vi "H1R_Ref_Pix_Subtract.vi"(9 "Num Ref Pix":i32=5, 11 "Orig Array":i32[][](array[numeric])=array1024x1024[1048576 elements]) -> (3 "Sub Array":i32[][](array[numeric]))   [LabVIEW 2017]
panel:
  out "Q3 avg":dbl=-0.8184616088867186
  out "Q3 RMS":dbl=19.25740971624928
  out "Q4 avg":dbl=1.3942337036132815
  out "Q4 RMS":dbl=26.97344260258525
  out "Q1 RMS":dbl=21.389760464347606
  out "Q1 avg":dbl=2.3578338623046875
  out "Q2  RMS":dbl=28.329968380841386
  out "Q2 avg":dbl=0.05986480712890625
  out "mean before":dbl=0.1424398422241211
  out "RMS before":dbl=23.67379491089448
  out "mean a fter":dbl=0.7448520660400391
  out "RMS  after":dbl=24.28217603569673
  out "IMAGE 2":i32[][](graph)
  out "IMAGE":i32[][](graph)
  in  "Array side Q3":u16(ring)=2 items=["Left", "Bottom", "Right", "Top"]
  in  "Array side Q4":u16(ring)=2 items=["Left", "Bottom", "Right", "Top"]
  in  "Array side Q1":u16(ring) items=["Left", "Bottom", "Right", "Top"]
  in  "Array side Q2":u16(ring) items=["Left", "Bottom", "Right", "Top"]
  # "right"
  # "left"
  # "left"
  # "right"
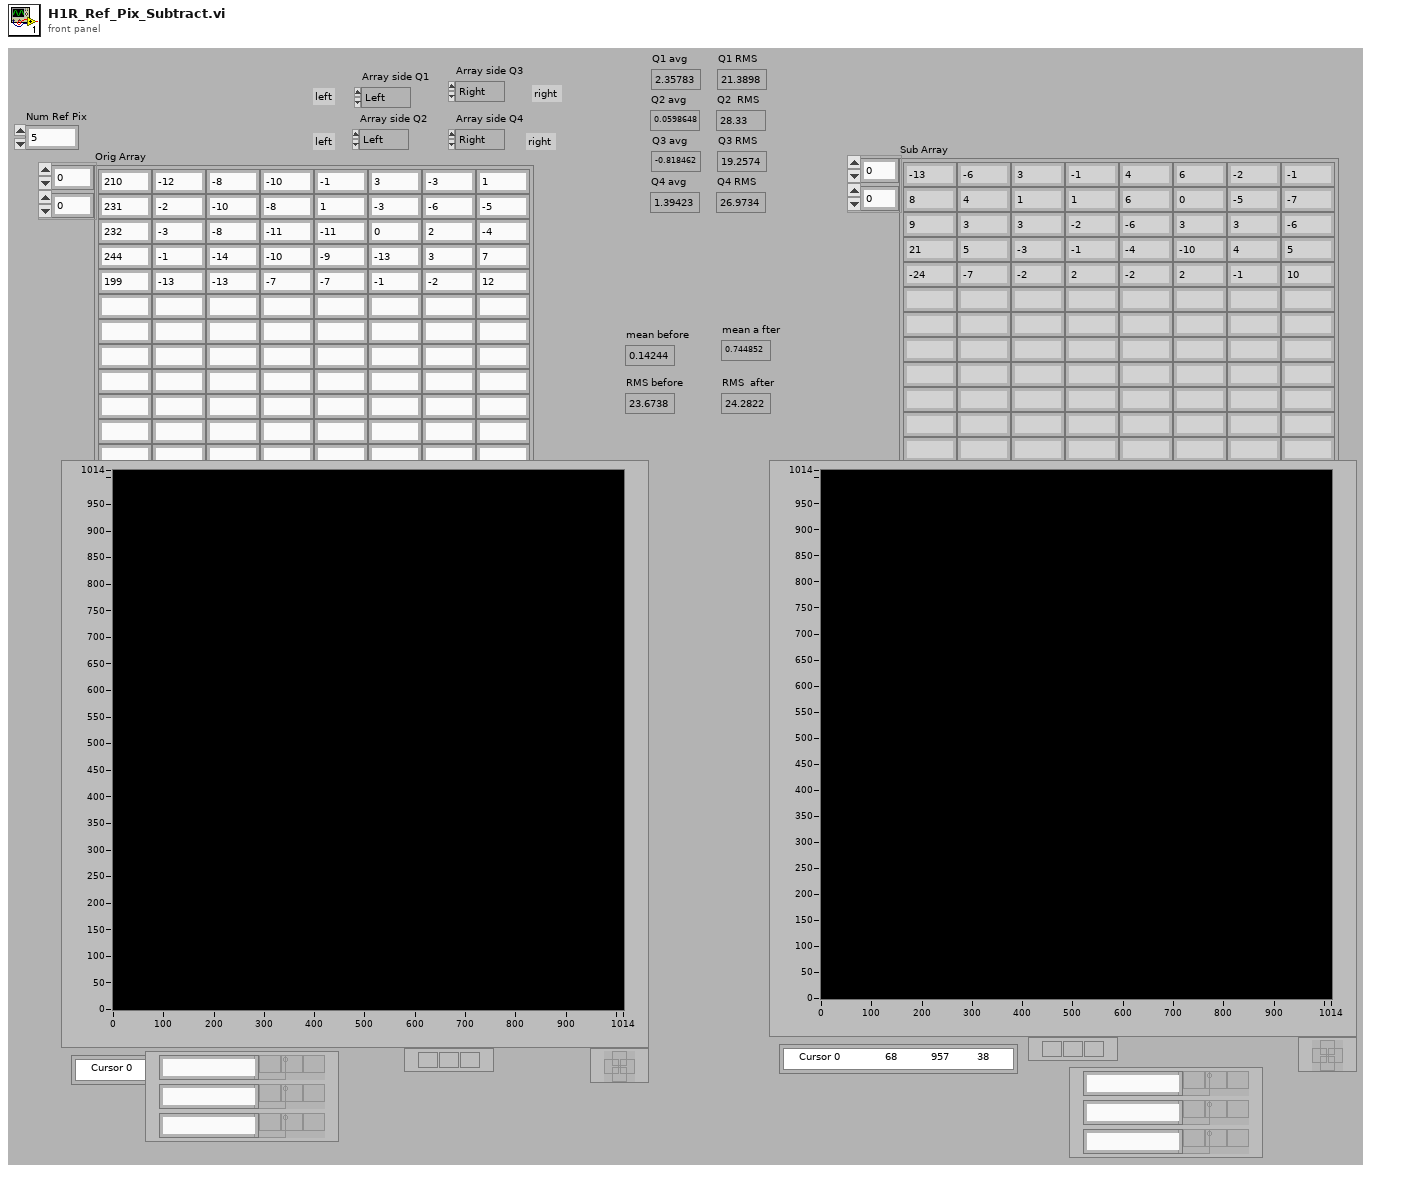
[diagram p1: front panel]
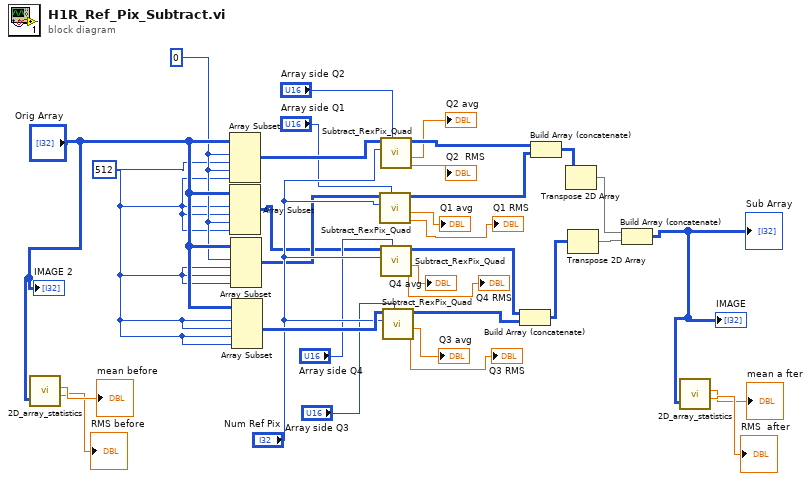
[diagram p0: block diagram]
diagram:
  w4 = 0
  w1 = 512
  n1 = call <userlib>:"2D_array_statistics.vi"("Array"="Orig Array") -> ("mean 2"=→"mean before":dbl, "RMS 2"=→"RMS before":dbl)  [unwired: 2 in, 2 out]
  n2 = Array Subset(array="Orig Array", index (row)=w4, length (row)=w1, index (col)=w4, length (col)=w1) -> (w29:i32[][])
  n3 = Array Subset(array="Orig Array", index (row)=w1, length (row)=w1, index (col)=w4, length (col)=w1) -> (w2:i32[][])
  n4 = Array Subset(array="Orig Array", index (row)=w4, length (row)=w1, index (col)=w1, length (col)=w1) -> (w3:i32[][])
  n5 = Array Subset(array="Orig Array", index (row)=w1, length (row)=w1, index (col)=w1, length (col)=w1) -> (w27:i32[][])
  n6 = call <userlib>:"Subtract_RexPix_Quad.vi"("Array side"="Array side Q1", "Num Ref Pix"="Num Ref Pix", "Quad array"=w3) -> ("RMS 2"=→"Q1 RMS":dbl, "mean 2"=→"Q1 avg":dbl, "Quad array subtracted ref pixs"=w25:i32[][])  [unwired: 5 in, 1 out]
  n7 = call <userlib>:"Subtract_RexPix_Quad.vi"("Array side"="Array side Q2", "Num Ref Pix"="Num Ref Pix", "Quad array"=w29) -> ("RMS 2"=→"Q2  RMS":dbl, "mean 2"=→"Q2 avg":dbl, "Quad array subtracted ref pixs"=w28:i32[][])  [unwired: 5 in, 1 out]
  n8 = call <userlib>:"Subtract_RexPix_Quad.vi"("Array side"="Array side Q4", "Num Ref Pix"="Num Ref Pix", "Quad array"=w2) -> ("RMS 2"=→"Q4 RMS":dbl, "mean 2"=→"Q4 avg":dbl, "Quad array subtracted ref pixs"=w24:i32[][])  [unwired: 5 in, 1 out]
  n9 = call <userlib>:"Subtract_RexPix_Quad.vi"("Array side"="Array side Q3", "Num Ref Pix"="Num Ref Pix", "Quad array"=w27) -> ("RMS 2"=→"Q3 RMS":dbl, "mean 2"=→"Q3 avg":dbl, "Quad array subtracted ref pixs"=w23:i32[][])  [unwired: 5 in, 1 out]
  n10 = Build Array (concatenate)(w24, w23) -> (w30:i32[][])
  n11 = Build Array (concatenate)(w28, w25) -> (w31:i32[][])
  n12 = Transpose 2D Array(2D array=w31) -> (transposed array=w32:i32[][])
  n13 = Transpose 2D Array(2D array=w30) -> (transposed array=w33:i32[][])
  n14 = Build Array (concatenate)(w32, w33) -> (w13:i32[][])
  "Sub Array" <- w13
  "IMAGE" <- w13
  n15 = call <userlib>:"2D_array_statistics.vi"("Array"=w13) -> ("mean 2"=→"mean a fter":dbl, "RMS 2"=→"RMS  after":dbl)  [unwired: 2 in, 2 out]
  "IMAGE 2" <- "Orig Array"
